vi "DeltaSigma.vi"() -> ()   [LabVIEW 2019]
uses:
  MeasSNRResults.ctl
  <vilib>/imath/engines/lvmath2/RunTimeEngine/NodeEndStatement/NIMS_NodeEndStatement_Output.vi
  <instcachedir>/0/NIMS_NodeEndStatement_Output_53EC0D466D134D7ABD903AC30B43404B.lvgen/NIMS_NodeEndStatement_Output_53EC0D466D134D7ABD903AC30B43404B_009.vi
  <instcachedir>/0/NIMS_NodeEndStatement_Output_53EC0D466D134D7ABD903AC30B43404B.lvgen/NIMS_NodeEndStatement_Output_53EC0D466D134D7ABD903AC30B43404B_001.vi
  <vilib>/imath/engines/lvmath2/RunTimeEngine/ErrorHandling/NIMS_Finalize Error.vi
  <vilib>/express/express analysis/Spectral/Block/exnSpectralBlock spectral measurements RMS poly.vi
  <vilib>/express/express analysis/Spectral/Block/exnSpectralBlock spectral measurements RMS array WFM.vi
  <vilib>/express/express analysis/Spectral/XNode/ExpressSpectralMeasurementsBlockNode.xnode
  <vilib>/measure/NI_MABase.lvlib
panel:
  out "ENOB vs D":cluster{"Y":dbl[], "Y":dbl[]}[](graph)=[{"Y"=[8.0, 16.0, 32.0, 64.0, 128.0, 256.0, 512.0], "Y"=[5.145136813912571, 7.691349281783459, 10.204082538184425, 12.719089748939503, 15.247718325665467, 17.666697780298676, 20.23980385820135]}, {"Y"=[8.0, 16.0, 32.0, 64.0, 128.0, 256.0, 512.0], "Y"=[5.421342779877434, 7.960368018712287, 10.50151763616172, 13.0204318460279, 15.569556029089421, 17.861821048518934, 19.702612468160403]}, {"Y"=[8.0, 16.0, 32.0, 64.0, 128.0, 256.0, 512.0], "Y"=[6.357142857142857, 8.857142857142858, 11.357142857142856, 13.857142857142856, 16.357142857142854, 18.857142857142854, 21.357142857142858]}]
  out "SNR vs D":cluster{"Y":dbl[], "Y":dbl[]}[](graph)=[{"Y"=[8.0, 16.0, 32.0, 64.0, 128.0, 256.0, 512.0], "Y"=[32.733723619753675, 48.061922676336415, 63.188576879870226, 78.3289202886158, 93.5512643205061, 108.11352063739803, 123.60361922637212]}, {"Y"=[8.0, 16.0, 32.0, 64.0, 128.0, 256.0, 512.0], "Y"=[34.39648353486215, 49.68141547264796, 64.97913616969355, 80.14299971308796, 95.48872729511831, 109.28816271208399, 120.36972705832562]}, {"Y"=[8.0, 16.0, 32.0, 64.0, 128.0, 256.0, 512.0], "Y"=[40.029999999999994, 55.08, 70.13, 85.17999999999999, 100.22999999999999, 115.27999999999999, 130.32999999999998]}]
  out "decimation factor":dbl=512.0
  out "Time Domain":waveform(dbl)[](graph)=[{"t0"=timestamp(0 s since 1904-01-01), "dt"=9.765625e-08, "Y"=array[2000000 elements]}, {"t0"=timestamp(0 s since 1904-01-01), "dt"=5e-05, "Y"=array[3907 elements]}] caption="Histogram"
  out "Frequency Domain":cluster{"f0":dbl, "df":dbl, "magnitude":dbl[]}[](graph)=[{"f0"=0.0, "df"=5.12, "magnitude"=array[1000000 elements]}, {"f0"=0.0, "df"=5.1190171487074485, "magnitude"=array[1954 elements]}] caption="Histogram"
  out "Decimation Results":T1[](array[typedef])=[{"VSignalRMS"=0.06817501546641716, "VNoiseRMS"=0.013479097831025933, "SNR(dB)"=14.079288394286163, "NumBits"=2.046393420977768, "SNRFS(dB)"=34.39648353486215, "NumBitsFS"=5.421342779877434}, {"VSignalRMS"=0.06920374460428923, "VNoiseRMS"=0.0023196060271958568, "SNR(dB)"=29.494307323330613, "NumBits"=4.607027794573192, "SNRFS(dB)"=49.68141547264796, "NumBitsFS"=7.960368018712287}, {"VSignalRMS"=0.07315266059326452, "VNoiseRMS"=0.0003985916473875562, "SNR(dB)"=45.274038650791795, "NumBits"=7.228245623055116, "SNRFS(dB)"=64.97913616969355, "NumBitsFS"=10.50151763616172}, {"VSignalRMS"=0.07392105470925868, "VNoiseRMS"=6.955606689936567e-05, "SNR(dB)"=60.52866276555516, "NumBits"=9.762236339793217, "SNRFS(dB)"=80.14299971308796, "NumBitsFS"=13.0204318460279}, {"VSignalRMS"=0.07150176585882292, "VNoiseRMS"=1.18863533737053e-05, "SNR(dB)"=75.58536260338046, "NumBits"=12.263349269664529, "SNRFS(dB)"=95.48872729511831, "NumBitsFS"=15.569556029089421}, {"VSignalRMS"=0.07115561650057928, "VNoiseRMS"=2.4270396231910517e-06, "SNR(dB)"=89.3426463843793, "NumBits"=14.548612356209185, "SNRFS(dB)"=109.28816271208399, "NumBitsFS"=17.861821048518934}, {"VSignalRMS"=0.06936052300883386, "VNoiseRMS"=6.776394000046381e-07, "SNR(dB)"=100.20227420000157, "NumBits"=16.352537242525177, "SNRFS(dB)"=120.36972705832562, "NumBitsFS"=19.702612468160403}] {"SNRFS(dB)" format="%_3p"; "NumBitsFS" format="%.1f"; "NumBits" format="%.1f"; "SNR(dB)" format="%_3p"; "VNoiseRMS" format="%#_3p"; "VSignalRMS" format="%#_3p"}
  out "Expected Results":T1[](array[typedef])=[{"VSignalRMS"=0.07071067811865475, "VNoiseRMS"=0.00704668733668855, "SNR(dB)"=20.029999999999994, "NumBits"=3.0348837209302317, "SNRFS(dB)"=40.029999999999994, "NumBitsFS"=6.357142857142857}, {"VSignalRMS"=0.07071067811865475, "VNoiseRMS"=0.0012459052107059259, "SNR(dB)"=35.08, "NumBits"=5.534883720930233, "SNRFS(dB)"=55.08, "NumBitsFS"=8.857142857142858}, {"VSignalRMS"=0.07071067811865475, "VNoiseRMS"=0.00022028503889795714, "SNR(dB)"=50.129999999999995, "NumBits"=8.034883720930234, "SNRFS(dB)"=70.13, "NumBitsFS"=11.357142857142856}, {"VSignalRMS"=0.07071067811865475, "VNoiseRMS"=3.894798572580023e-05, "SNR(dB)"=65.17999999999999, "NumBits"=10.534883720930232, "SNRFS(dB)"=85.17999999999999, "NumBitsFS"=13.857142857142856}, {"VSignalRMS"=0.07071067811865475, "VNoiseRMS"=6.886285149850018e-06, "SNR(dB)"=80.22999999999999, "NumBits"=13.034883720930232, "SNRFS(dB)"=100.22999999999999, "NumBitsFS"=16.357142857142854}, {"VSignalRMS"=0.07071067811865475, "VNoiseRMS"=1.2175449456846246e-06, "SNR(dB)"=95.27999999999999, "NumBits"=15.53488372093023, "SNRFS(dB)"=115.27999999999999, "NumBitsFS"=18.857142857142854}, {"VSignalRMS"=0.07071067811865475, "VNoiseRMS"=2.1527073923078286e-07, "SNR(dB)"=110.32999999999998, "NumBits"=18.03488372093023, "SNRFS(dB)"=130.32999999999998, "NumBitsFS"=21.357142857142858}] {"SNRFS(dB)" format="%_3p"; "NumBitsFS" format="%.1f"; "NumBits" format="%.1f"; "SNR(dB)" format="%_3p"; "VNoiseRMS" format="%#_3p"; "VSignalRMS" format="%#_3p"}
  out "Brick Wall (Modulation) Results":T1[](array[typedef])=[{"VSignalRMS"=0.07071096293295302, "VNoiseRMS"=0.016322956422196916, "SNR(dB)"=12.733758605425514, "NumBits"=1.8228834892733414, "SNRFS(dB)"=32.733723619753675, "NumBitsFS"=5.145136813912571}, {"VSignalRMS"=0.07071096293295302, "VNoiseRMS"=0.002795045411675449, "SNR(dB)"=28.061957662008254, "NumBits"=4.3690959571442285, "SNRFS(dB)"=48.061922676336415, "NumBitsFS"=7.691349281783459}, {"VSignalRMS"=0.07071096293295302, "VNoiseRMS"=0.0004898421562607017, "SNR(dB)"=43.18861186554206, "NumBits"=6.881829213545193, "SNRFS(dB)"=63.188576879870226, "NumBitsFS"=10.204082538184425}, {"VSignalRMS"=0.07071096293295302, "VNoiseRMS"=8.571147871846502e-05, "SNR(dB)"=58.32895527428764, "NumBits"=9.396836424300274, "SNRFS(dB)"=78.3289202886158, "NumBitsFS"=12.719089748939503}, {"VSignalRMS"=0.07071096293295302, "VNoiseRMS"=1.4856680581973776e-05, "SNR(dB)"=73.55129930617795, "NumBits"=11.925465001026238, "SNRFS(dB)"=93.5512643205061, "NumBitsFS"=15.247718325665467}, {"VSignalRMS"=0.07071096293295302, "VNoiseRMS"=2.77849084599016e-06, "SNR(dB)"=88.11355562306986, "NumBits"=14.344444455659445, "SNRFS(dB)"=108.11352063739803, "NumBitsFS"=17.666697780298676}, {"VSignalRMS"=0.07071096293295302, "VNoiseRMS"=4.6698619356377516e-07, "SNR(dB)"=103.60365421204395, "NumBits"=16.917550533562117, "SNRFS(dB)"=123.60361922637212, "NumBitsFS"=20.23980385820135}] {"SNRFS(dB)" format="%_3p"; "NumBitsFS" format="%.1f"; "NumBits" format="%.1f"; "SNR(dB)" format="%_3p"; "VNoiseRMS" format="%#_3p"; "VSignalRMS" format="%#_3p"}
  in  "Vref":dbl=1.0
  in  "sampling info":cluster{"Fs":dbl, "#s":dbl}={"Fs"=10240000.0, "#s"=2000000.0} {"Fs" format="%.2p"}
  in  "amplitude":dbl=0.1 format="%0.2p"
  in  "frequency":dbl=5001.0 format="%0.2p"
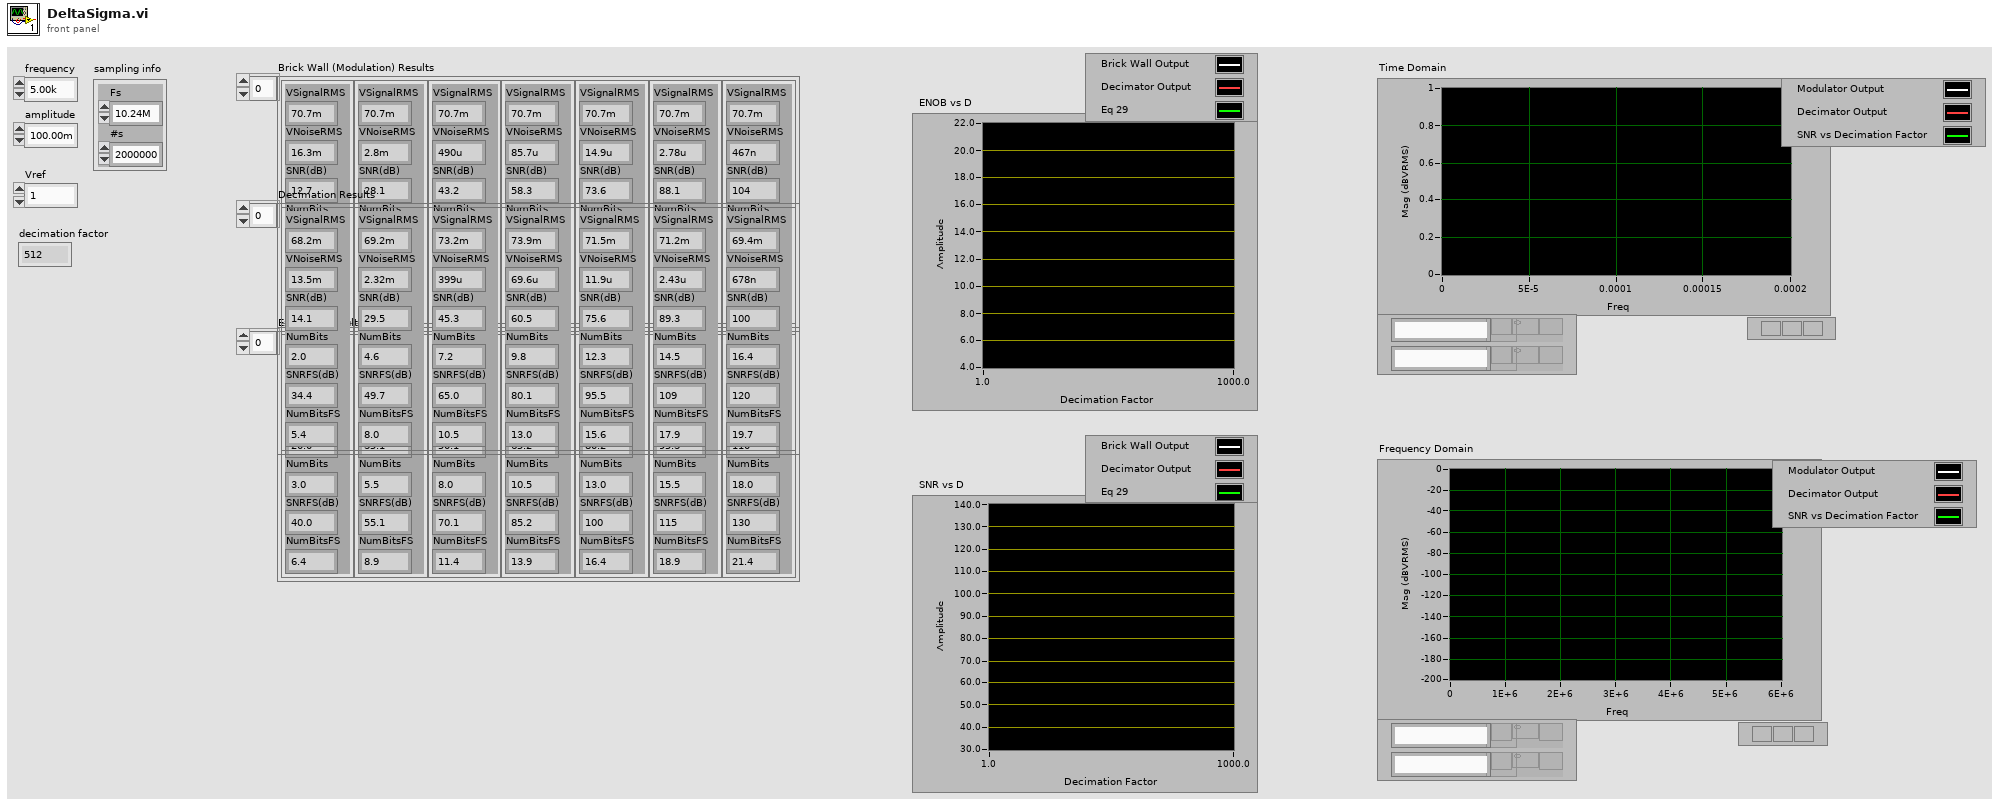
[diagram p1: front panel]
types:
  T1 = typedef "MeasSNRResults.ctl" = cluster{"VSignalRMS":dbl, "VNoiseRMS":dbl, "SNR(dB)":dbl, "NumBits":dbl, "SNRFS(dB)":dbl, "NumBitsFS":dbl}
  T2 = enum16{"Sine Wave", "Triangle Wave", "Square Wave", "Sawtooth Wave"}
  T3 = cluster{"averaging mode":u16, "weighting mode":u16, "number of averages":u32}
  T4 = cluster{"dB On (F)":bool, "unwrap phase (F)":bool, "convert to degree (F)":bool}
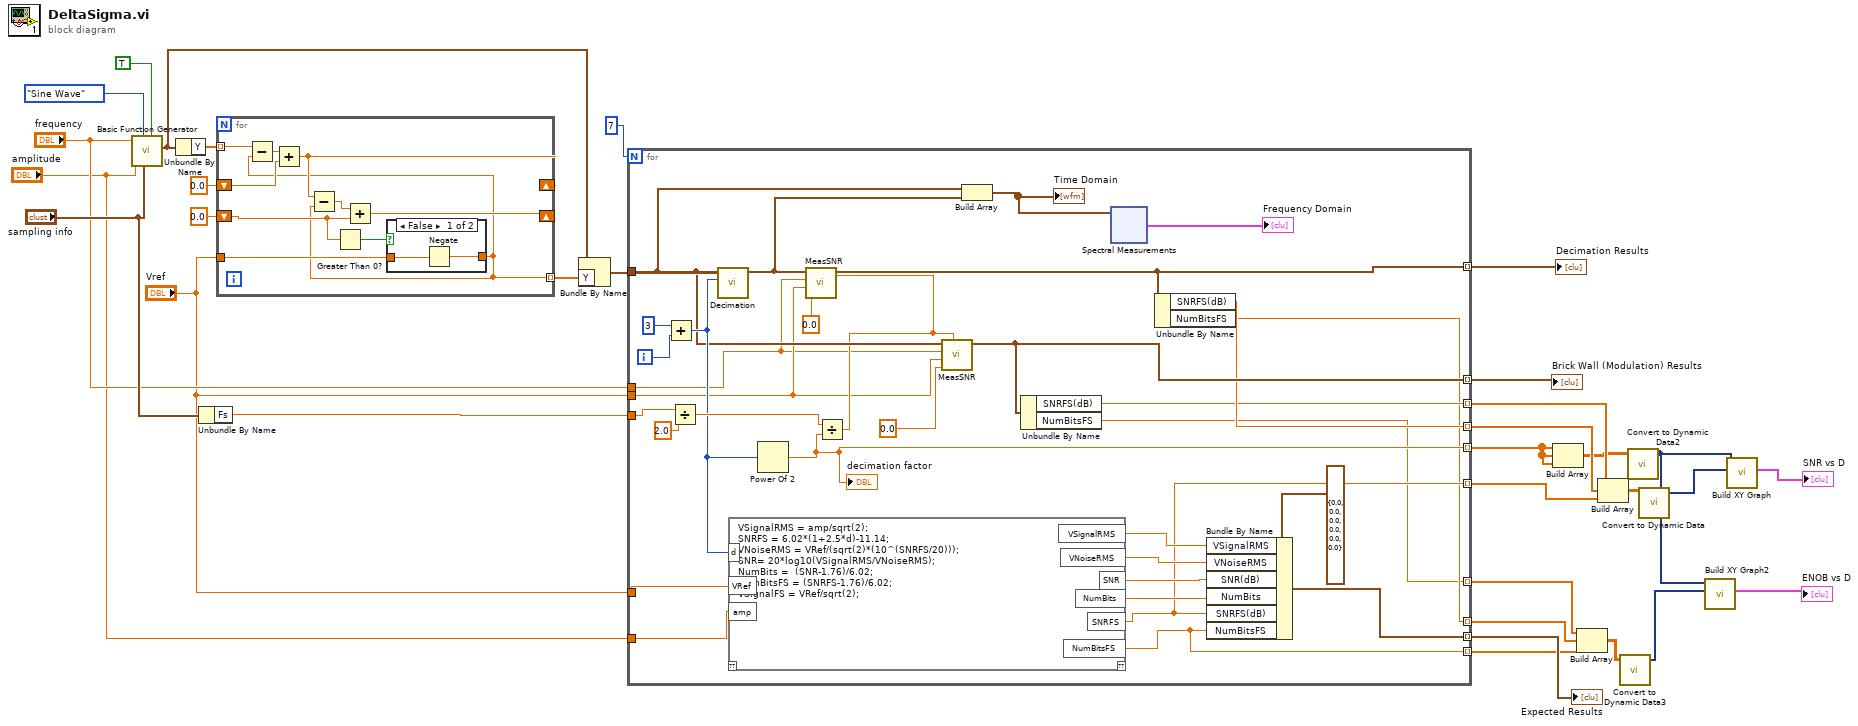
[diagram p0: block diagram]
diagram:
  n1 = call <vilib>:"Basic Function Generator.vi"("reset signal"=TRUE, "sampling info"="sampling info", "signal type"=T2."Sine Wave", "amplitude"="amplitude", "frequency"="frequency") -> ("signal out"=w29:waveform(dbl))  [unwired: 4 in, 2 out]
  n2 = Unbundle By Name(w29) -> ("Y"=w30:dbl[])
  n3 = Unbundle By Name("sampling info") -> ("Fs"=w25:dbl)
  n4 = for {
    tunnel: w30 -> [w41] mode=indexing
    shift-right: [w37] -> _
    shift-left: 0.0 -> [w34]
    shift-right: [w39] -> _
    shift-left: 0.0 -> [w40]
    tunnel: "Vref" -> [w35]
    tunnel: [w33] -> w1 mode=indexing
    n5 = Greater Than 0?(x=w34) -> (x > 0?=w36:bool)
    n6 = case shown="False" w36 {
      tunnel: [w44 w45] -> w33
      tunnel: w35 -> [w43 w45]
      frame False {
        n7 = Negate(x=w43) -> (-x=w44:dbl)
      }
      frame True {
      }
    }
    n8 = Subtract(x=w41, y=w33) -> (x-y=w42:dbl)
    n9 = Add(x=w42, y=w40) -> (x+y=w39:dbl)
    n10 = Subtract(x=w39, y=w33) -> (x-y=w38:dbl)
    n11 = Add(x=w38, y=w34) -> (x+y=w37:dbl)
  }
  n12 = Bundle By Name(cluster=w29, "Y"=w1) -> (w19:waveform(dbl))
  n13 = for {
    N: 7 -> [_]
    tunnel: w19 -> [w55]
    tunnel: w25 -> [w76]
    tunnel: "frequency" -> [w46]
    tunnel: "Vref" -> [w47]
    tunnel: [w54] -> w23 mode=indexing
    tunnel: "Vref" -> [w70]
    tunnel: "amplitude" -> [w68]
    tunnel: [w64] -> w21 mode=indexing
    tunnel: [w57] -> w20 mode=indexing
    tunnel: [w59] -> w5 mode=indexing
    tunnel: [w58] -> w16 mode=indexing
    tunnel: [w56] -> w11 mode=indexing
    tunnel: [w53] -> w15 mode=indexing
    tunnel: [w52] -> w14 mode=indexing
    tunnel: [w51] -> w10 mode=indexing
    tunnel: [w50] -> w9 mode=indexing
    i -> [w60]
    n14 = Add(x=3, y=w60) -> (x+y=w72:i32)
    n15 = Divide(x=w76, y=2.0) -> (x/y=w74:dbl)
    n16 = call "Decimation.vi"("d"=w72, "signal in"=w55) -> ("output waveform"=w63:waveform(dbl))  [unwired: 9 in]
    n17 = mathscript code="VSignalRMS = amp/sqrt(2);\nSNRFS = 6.02*(1+2.5*d)-11.14;\nVNoiseRMS = VRef/(sqrt(2)*(10^(SNRFS/20)));\nSNR= 20*log10(VSignalRMS/VNoiseRMS); \nNumBits =  (SNR-1.76)/6.02;\nNumBitsFS = (SNRFS-1.76)/6.02;\nVSignalFS = VRef/sqrt(2);"("d"=w72, "VRef"=w70, "amp"=w68) -> ("VNoiseRMS"=w69:cdb, "SNRFS"=w58:dbl, "NumBitsFS"=w56:dbl, "VSignalRMS"=w67:cdb, "SNR"=w66:cdb, "NumBits"=w65:cdb)  [unwired: 1 in, 1 out]
    n18 = Power Of 2(x=w72) -> (2^x=w59:dbl)
    "decimation factor" <- w59
    n19 = Divide(x=w74, y=w59) -> (x/y=w49:dbl)
    n20 = call "MeasSNR.vi"("UpperNoiseBW"=w49, "LowerNoiseBW"=0.0, "VRef"=w47, "FSignal"=w46, "Input"=w63) -> ("MeasSNRResults"=w57:T1)  [unwired: 5 in, 1 out]
    n21 = call "MeasSNR.vi"("UpperNoiseBW"=w49, "LowerNoiseBW"=0.0, "VRef"=w47, "FSignal"=w46, "Input"=w55) -> ("MeasSNRResults"=w54:T1)  [unwired: 5 in, 1 out]
    n22 = Build Array(w55, w63) -> (w62:waveform(dbl)[])
    "Time Domain" <- w62
    n23 = Unbundle By Name(w54) -> ("SNRFS(dB)"=w52:dbl, "NumBitsFS"=w50:dbl)
    n24 = xnode "Spectral Measurements"("Signals"=w62) -> ("FFT - (RMS)"=→"Frequency Domain":cluster{"f0":dbl, "df":dbl, "magnitude":dbl[]}[])  [unwired: 1 in, 2 out]
    n25 = Unbundle By Name(w57) -> ("SNRFS(dB)"=w53:dbl, "NumBitsFS"=w51:dbl)
    n26 = Bundle By Name(cluster=T1 {"VSignalRMS"=0.0, "VNoiseRMS"=0.0, "SNR(dB)"=0.0, "NumBits"=0.0, "SNRFS(dB)"=0.0, "NumBitsFS"=0.0} ("MeasSNRResults"), "VSignalRMS"=w67, "VNoiseRMS"=w69, "SNR(dB)"=w66, "NumBits"=w65, "SNRFS(dB)"=w58, "NumBitsFS"=w56) -> (w64:T1)
  }
  "Brick Wall (Modulation) Results" <- w23
  "Expected Results" <- w21
  "Decimation Results" <- w20
  n27 = Build Array(w5, w5, w5) -> (w4:dbl[][])
  n28 = Build Array(w9, w10, w11) -> (w8:dbl[][])
  n29 = Build Array(w14, w15, w16) -> (w13:dbl[][])
  n30 = call "Convert to Dynamic Data3"("2D Array"=w8) -> ("Dynamic Data Type"=w7:dynamicdata)  [unwired: 3 in]
  n31 = call "Convert to Dynamic Data2"("2D Array"=w4) -> ("Dynamic Data Type"=w3:dynamicdata)  [unwired: 3 in]
  n32 = call "Convert to Dynamic Data"("2D Array"=w13) -> ("Dynamic Data Type"=w12:dynamicdata)  [unwired: 3 in]
  n33 = call "Build XY Graph2"("Y Input"=w7, "X Input"=w3) -> ("XY Graph"=→"ENOB vs D":cluster{"X":dbl[], "Y":dbl[]}[])  [unwired: 8 in, 1 out]
  n34 = call "Build XY Graph"("Y Input"=w12, "X Input"=w3) -> ("XY Graph"=→"SNR vs D":cluster{"X":dbl[], "Y":dbl[]}[])  [unwired: 8 in, 1 out]
